vi "HFRR ADV v043.vi"() -> ()   [LabVIEW 2025] (continued)
                n2741 = Multiply(x=w3264, y=w3250) -> (x*y=w3256:dbl)
                n2742 = Subtract(x=w3257, y=w3267) -> (x-y=w3259:dbl)
                n2743 = local read "Save"() -> (w3260:bool)
                n2744 = Add(x=w3259, y=w3256) -> (x+y=w3243:dbl)
                "Elapsed time 3" <- w3243
                n2745 = And(x=w3245, y=w3260) -> (x .and. y?=w3258:bool)
                n2746 = Divide(x=w3243, y=60.0) -> (x/y=w3254:dbl)
                n2747 = local read "Test \nStatus"() -> (w3244:bool)
                n2748 = local read "clk"() -> (w3251:dbl)
                n2749 = Equal?(x=w3251, y=10.0) -> (x = y?=w3253:bool)
                n2750 = case shown="True" w3258 {
                  tunnel: w3257 -> [_ w3384]
                  tunnel: [FALSE ("Boolean 2") TRUE ("Boolean 2")] -> _
                  frame False {
                  }
                  frame True {
                    w3338 = ";" ("Substring")
                    # "Pid out/\nFreq response value"
                    n2751 = local write "act save time"(w3384) -> ()
                    n2752 = local read "FILE"() -> (w3332:string)
                    n2753 = call "file check.vi"("file name in"=w3332) -> ("error out"=w3335:errorcluster, "file name out"=w3330:string)  [unwired: 9 in]
                    n2754 = local read "LVDT STROKE"() -> (w3327:dbl)
                    n2755 = local read "Add up Stroke"() -> (w3325:dbl)
                    n2756 = call "FILE PATH CREATION.vi"("error in"=w3335, "FILE NAME :"=w3330) -> ("FILE OUT"=w3333:path)  [unwired: 8 in, 1 out]
                    n2757 = local read "STROKE Initialize"() -> (w3320:bool)
                    n2758 = Concatenate Strings(w3330, ".dgf" ("Substring")) -> (w3334:string)
                    n2759 = Subtract(x=w3327, y=w3325) -> (x-y=w3326:dbl)
                    n2760 = Absolute Value(x=w3326) -> (abs(x)=w3323:dbl)
                    n2761 = local read "FF 2"() -> (→"Frictional Force ( N )" →"Frictional Force ( N )":dbl)
                    n2762 = Build Path(base path=w3333, name or relative path=w3334) -> (appended path=w3329:path)
                    n2763 = flat-sequence {
                      tunnel: w3323 -> [w3389]
                      tunnel: [w3388] -> w3321
                      tunnel: w3320 -> [w3386]
                      tunnel: [w3391] -> w3322
                      tunnel: w3321 -> [w3391]
                      frame #0 {
                        n2764 = call <vilib>:"Mean PtByPt.vi"("x"=w3389, "sample length"="STROKE FILTER", "initialize"=w3386) -> ("mean"=w3388:dbl)  [unwired: 1 in, 1 out]
                      }
                      frame #1 {
                        "STROKE Initialize" <- FALSE ("STROKE Initialize")
                      }
                    }
                    n2765 = local read "COF 2"() -> (w3343:dbl)
                    "Coefficient of Friction" <- w3343
                    "COF 4" <- w3343
                    "Coefficient of Friction" <- w3343
                    n2766 = local read "TEMP"() -> (w3346:dbl)
                    "Temperature ( Deg C )" <- w3346
                    n2767 = local read "Humidity ( %RH )"() -> (w3345:dbl)
                    n2768 = local read "Frequency ( Hz )"() -> (w3352:dbl)
                    n2769 = local read "LVDT STROKE DISPLAY"() -> (w3324:dbl)
                    n2770 = local read "Elapsed time"() -> (w3377:dbl)
                    n2771 = local read "AIR TEMP"() -> (w3350:dbl)
                    n2772 = local read "PID-out"() -> (w3355:dbl)
                    n2773 = local write "Temperature ( Deg C )"(w3346) -> ()
                    n2774 = Number To Fractional String(number=w3324, width (-)=i16 9 ("precision (6)"), precision (6)=i16 6) -> (F-format string=w3370:string)  [unwired: 1 in]
                    n2775 = Number To Fractional String(number=w3350, width (-)=i16 9 ("precision (6)"), precision (6)=i16 3) -> (F-format string=w3369:string)  [unwired: 1 in]
                    n2776 = Number To Fractional String(number=w3346, width (-)=i16 9 ("precision (6)"), precision (6)=i16 3) -> (F-format string=w3366:string)  [unwired: 1 in]
                    n2777 = Number To Fractional String(number=w3345, width (-)=i16 9 ("precision (6)"), precision (6)=i16 3) -> (F-format string=w3363:string)  [unwired: 1 in]
                    n2778 = Number To Fractional String(number=0.0, width (-)=i16 9 ("precision (6)"), precision (6)=i16 3) -> (F-format string=w3360:string)  [unwired: 1 in]
                    n2779 = Number To Fractional String(number=w3355, width (-)=i16 9 ("precision (6)"), precision (6)=i16 3) -> (F-format string=w3356:string)  [unwired: 1 in]
                    n2780 = Number To Fractional String(number=w3352, width (-)=i16 9 ("precision (6)"), precision (6)=i16 3) -> (F-format string=w3351:string)  [unwired: 1 in]
                    n2781 = Number To Fractional String(number=w3343, width (-)=i16 9 ("precision (6)"), precision (6)=i16 6) -> (F-format string=w3378:string)  [unwired: 1 in]
                    n2782 = Number To Fractional String(number=w3377, width (-)=i16 14 ("precision (6)"), precision (6)=i16 3) -> (F-format string=w3379:string)  [unwired: 1 in]
                    n2783 = Bundle("y"=1.02, "LVDT STROKE DISPLAY"=w3324, "y"=0.98) -> (w3344:T30)  [unwired: 1 in]
                    n2784 = Number To Fractional String(number="Ambient Humidity :", width (-)=i16 9 ("precision (6)"), precision (6)=i16 6) -> (F-format string=w3336:string)  [unwired: 1 in]
                    n2785 = local read "RUN"() -> (w3342:bool)
                    n2786 = case shown="True" w3342 {
                      tunnel: w3344 -> [_ w3395]
                      tunnel: w3324 -> [_ w3394]
                      tunnel: w3324 -> [_ w3392]
                      tunnel: w3324 -> [_ w3393]
                      frame False {
                      }
                      frame True {
                        "Stroke ( mm )" <- w3395
                        "Stroke ( mm )" <- w3395
                        "Stroke 4" <- w3394
                        "Stroke 3" <- w3392
                        "Stroke 2" <- w3393
                        "measured_stroke" <- w3392
                      }
                    }
                    n2787 = Concatenate Strings(w3379, w3338, w3378, w3338, w3370, w3338, w3369, w3338, w3366, w3338, w3363, w3338, w3360, w3338, w3356, w3338, w3351, w3338, w3336, "\r") -> (w3376:string)
                    n2788 = call <vilib>:"Write Characters To File.vi"("append to file? (new file:F)"=TRUE, "character string"=w3376, "file path (dialog if empty)"=w3329) -> ()  [unwired: 2 in, 1 out]
                    "refresh flag" <- TRUE ("refresh flag")
                    "LVDT STROKE Actual" <- w3322
                  }
                }
                n2789 = case shown="True" w3244 {
                  tunnel: w3254 -> [_ w3280]
                  tunnel: w3259 -> [_ w3290]
                  tunnel: [0.0 w3286] -> _
                  tunnel: w3253 -> [_ w3285]
                  tunnel: [0.0 w3284] -> _
                  tunnel: w3243 -> [_ w3284]
                  tunnel: w3257 -> [w3273 _]
                  frame False {
                    n2790 = local write "acq timer"(w3273) -> ()
                    n2791 = local write "Test Duration Status"(0.0 ("Test Duration Status")) -> ()
                  }
                  frame True {
                    n2792 = local read "Set Hz"() -> (w3287:dbl)
                    n2793 = local write "Elapsed time"(w3280) -> ()
                    n2794 = local read "test time"() -> (w3279:dbl)
                    n2795 = Multiply(x=w3290, y=w3287) -> (x*y=w3289:dbl)
                    n2796 = case shown="False" w3285 {
                      tunnel: w3289 -> [w3291 _]
                      tunnel: [w3291 1.0] -> w3286
                      frame False {
                        n2797 = local write "Cycles elapsed"(w3291) -> ()
                      }
                      frame True {
                      }
                    }
                    n2798 = Greater?(x=w3280, y=w3279) -> (0:w3288:bool)
                    n2799 = Subtract(x=w3279, y=w3280) -> (x-y=w3278:dbl)
                    n2800 = Multiply(x=w3278, y=60.0) -> (x*y=w3277:dbl)
                    n2801 = local write "Time Remaining"(w3277) -> ()
                    n2802 = local write "Remaining Time"(w3277) -> ()
                    n2803 = case shown="True" w3288 {
                      frame False {
                      }
                      frame True {
                        n2804 = stacked-sequence {
                          frame #0 {
                            w3296 = T19."Enabled" ("Disabled")
                            w3295 = FALSE ("TEST FILE NAM,E SAVED")
                            w3297 = "" ("FILE")
                            w3298 = TRUE ("Visible")
                            n2805 = local write "Humidity"(FALSE ("Humidity")) -> ()
                            n2806 = local write "RUN"(FALSE ("OK Button 2")) -> ()
                            n2807 = local write "Heater Button"(FALSE ("Heater Button")) -> ()
                            n2808 = local write "Auto Start Test"(FALSE ("Auto Start Test")) -> ()
                            n2809 = local write "TestCompFlg"(TRUE ("StpFlg")) -> ()
                            n2810 = local read "Humidity ( %RH )"() -> (→"Rh After":dbl)
                            n2811 = property on="STOP 2" class="Bool (strict)"("Disabled"=u8 0) -> ()  [unwired: 2 in, 2 out]
                            n2812 = local read "EVENT LOG"() -> (w3303:string)
                            n2813 = call "Event Log.vi"("Content"="Test Completed", "EVENT LOG"=w3303) -> ("EVENT LOG"=w3302:string)  [unwired: 8 in, 1 out]
                            n2814 = property on="RUN" class="Bool (strict)"("Visible"=w3298) -> ()  [unwired: 2 in, 2 out]
                            n2815 = property on="Auto Start Test" class="Bool (strict)"("Visible"=w3298) -> ()  [unwired: 2 in, 2 out]
                            n2816 = local write "Batch Ref Num :"(w3297) -> ()
                            n2817 = local write "FILE"(w3297) -> ()
                            n2818 = local write "EVENT LOG"(w3302) -> ()
                            n2819 = local write "TEST FILE NAM,E SAVED"(w3295) -> ()
                            n2820 = local write "Fuel Discription :"(w3297) -> ()
                            n2821 = local write "START TEMP"(w3295) -> ()
                            n2822 = local write "Remarks :"(w3297) -> ()
                            n2823 = local write "Main Dashboard Buttons"(T1."Imaging" ("Main Dashboard Buttons")) -> ()
                            n2824 = local write "Main Tab"(T2."Adv Scar" ("Main Tab")) -> ()
                            n2825 = property on="FRICVALZ 2" class="Bool (strict)"("DisabledEnum"=w3296) -> ()  [unwired: 2 in, 2 out]
                            n2826 = property on="FRICVALZ 3" class="Bool (strict)"("DisabledEnum"=w3296) -> ()  [unwired: 2 in, 2 out]
                            n2827 = property on="FRICVALZ 4" class="Bool (strict)"("DisabledEnum"=w3296) -> ()  [unwired: 2 in, 2 out]
                          }
                          frame #1 {
                            n2828 = Wait (ms)(milliseconds to wait=u32 2000) -> ()  [unwired: 1 out]
                          }
                          frame #2 {
                            n2829 = local write "Due Write"("VC;0") -> ()
                          }
                          frame #3 {
                            n2830 = Wait (ms)(milliseconds to wait=u32 2000) -> ()  [unwired: 1 out]
                          }
                          frame #4 {
                            n2831 = local write "Due Write"("VC;0") -> ()
                          }
                          frame #5 {
                            n2832 = Wait (ms)(milliseconds to wait=u32 2000) -> ()  [unwired: 1 out]
                          }
                          frame #6 {
                            n2833 = local write "Due Write"("ST;0") -> ()
                          }
                          frame #7 {
                            n2834 = local write "measured_stroke"(0.0 ("measured_stroke")) -> ()
                            n2835 = Wait (ms)(milliseconds to wait=u32 1500) -> ()  [unwired: 1 out]
                          }
                          frame #8 {
                            n2836 = local write "Due Write"("HE;0") -> ()
                            n2837 = local write "Humidity 2"(TRUE ("Humidity")) -> ()
                          }
                        }
                      }
                    }
                    n2838 = Divide(x=w3280, y=w3279) -> (x/y=w3283:dbl)
                    n2839 = Multiply(x=w3283, y=100.0) -> (x*y=w3281:dbl)
                    n2840 = local write "Test Duration Status"(w3281) -> ()
                  }
                }
              }
              frame #2 {
                n2841 = case shown="True" "Heater Button" {
                  tunnel: [0.0 ("output") w3418] -> w3396
                  frame False {
                    w3399 = TRUE ("tmpchk")
                    n2842 = local read "TEMP"() -> (w3400:dbl)
                    n2843 = local write "Temp ini"(w3400) -> ()
                    n2844 = local write "Reset 4"(w3399) -> ()
                    n2845 = local write "tmpchk"(w3399) -> ()
                    n2846 = local write "reinit"(TRUE ("reinit")) -> ()
                    n2847 = local write "manual temp log"(TRUE ("manual temp log")) -> ()
                  }
                  frame True {
                    # "Logic to turn off\nthe heater when \ntemp is not rising.\nTime - 60 sec\nDelta t- 5°c"
                    n2848 = local read "Temp ini"() -> (w3407:dbl)
                    n2849 = local read "Auto Start Test"() -> (w3403:bool)
                    n2850 = Less?(x=w3407, y=53.0) -> (x < y?=w3405:bool)
                    n2851 = case shown="False" w3403 {
                      frame False {
                        n2852 = local read "Set Temp"() -> (w3427:dbl)
                        n2853 = local read "TEMP"() -> (w3426:dbl)
                        n2854 = Subtract(x=w3427, y=w3426) -> (x-y=w3425:dbl)
                        n2855 = Absolute Value(x=w3425) -> (abs(x)=w3424:dbl)
                        n2856 = Less?(x=w3424, y=0.5) -> (x < y?=w3422:bool)
                        n2857 = case shown="True" w3422 {
                          tunnel: "manual temp log" -> [_ w3428]
                          frame False {
                          }
                          frame True {
                            n2858 = case shown="True" w3428 {
                              selector: w3428 -> [_ w3429]
                              frame False {
                              }
                              frame True {
                                # "#Event log"
                                n2859 = Not(x=w3429) -> (.not. x?=w3430:bool)
                                n2860 = local write "manual temp log"(w3430) -> ()
                                n2861 = local read "EVENT LOG"() -> (w3433:string)
                                n2862 = call "Event Log.vi"("Content"="Target Temperature reached", "EVENT LOG"=w3433) -> ("EVENT LOG"=w3432:string)  [unwired: 8 in, 1 out]
                                n2863 = local write "EVENT LOG"(w3432) -> ()
                              }
                            }
                          }
                        }
                      }
                      frame True {
                        n2864 = local write "manual temp log"(TRUE ("manual temp log")) -> ()
                      }
                    }
                    n2865 = And(x="tmpchk", y=w3405) -> (x .and. y?=w3408:bool)
                    n2866 = case shown="True" w3408 {
                      frame False {
                      }
                      frame True {
                        n2867 = call "Elapsed Time8"("Time Target (s)"=300.0, "Reset"="Reset 4") -> ("Time has Elapsed"=w3435:bool)  [unwired: 10 in, 7 out]
                        n2868 = flat-sequence {
                          tunnel: w3435 -> [_]
                          frame #0 {
                            n2869 = local write "Reset 4"(FALSE ("Reset 4")) -> ()
                          }
                        }
                        n2870 = case shown="True" w3435 {
                          frame False {
                          }
                          frame True {
                            n2871 = local read "Temp ini"() -> (w3442:dbl)
                            n2872 = Add(x=w3442, y=5.0) -> (x+y=w3440:dbl)
                            n2873 = local read "TEMP"() -> (w3443:dbl)
                            n2874 = Greater?(x=w3443, y=w3440) -> (0:w3441:bool)
                            n2875 = case shown="False" w3441 {
                              frame False {
                                n2876 = local write "Heater Button"(FALSE ("Heater Button")) -> ()
                              }
                              frame True {
                                n2877 = local write "tmpchk"(FALSE ("tmpchk")) -> ()
                              }
                            }
                          }
                        }
                      }
                    }
                    n2878 = local read "Set Temp"() -> (w3416:dbl)
                    n2879 = local read "TEMP"() -> (w3410:dbl)
                    n2880 = call-poly <vilib>:"PID.vi"("reinitialize? (F)"="reinit", "dt (s)"=-1.0, "process variable"=w3410, "setpoint"=w3416) -> ("output"=w3413:dbl)  [unwired: 6 in, 1 out]
                    n2881 = Subtract(x=w3416, y=w3410) -> (x-y=w3417:dbl)
                    n2882 = Add(x=w3416, y=0.5) -> (x+y=w3414:dbl)
                    n2883 = Greater Or Equal?(x=w3410, y=w3414) -> ()  [unwired: 1 out]
                    n2884 = Select(t=0.0, s=FALSE, f=w3413) -> (s? t:f=w3412:dbl)
                    "PID output" <- w3412
                    n2885 = flat-sequence {
                      tunnel: w3412 -> [w3446]
                      tunnel: [w3446] -> w3418
                      frame #0 {
                        n2886 = local write "reinit"(FALSE ("reinit")) -> ()
                      }
                    }
                    n2887 = Bundle(w3417, "output"=w3412, "TEMP"=w3410) -> ()  [unwired: 1 in, 1 out]
                  }
                }
                "PID-out" <- w3396
              }
              frame #3 {
                n2888 = local read "TEMP"() -> (w3448:dbl)
                n2889 = Greater Or Equal?(x=w3448, y="Set Temp 2") -> (x >= y?=w3453:bool)
                n2890 = case shown="True" w3453 {
                  tunnel: [FALSE TRUE] -> w3451
                  frame False {
                  }
                  frame True {
                  }
                }
                "Status 13" <- w3451
                n2891 = And(x=w3451, y="trip1 8") -> (x .and. y?=w3450:bool)
                n2892 = case shown="True" w3450 {
                  frame False {
                    n2893 = local write "Heater Trip Temp"(TRUE ("Heater Trip Temp")) -> ()
                  }
                  frame True {
                    w3456 = FALSE ("OK Button 2")
                    n2894 = case shown="True" "Heater Trip Temp" {
                      selector: "Heater Trip Temp" -> [_ w3458]
                      frame False {
                      }
                      frame True {
                        n2895 = Not(x=w3458) -> (.not. x?=w3457:bool)
                        n2896 = local read "EVENT LOG"() -> (w3461:string)
                        n2897 = local write "Heater Trip Temp"(w3457) -> ()
                        n2898 = call "Event Log.vi"("Content"="Heater Trip", "EVENT LOG"=w3461) -> ("EVENT LOG"=w3460:string)  [unwired: 8 in, 1 out]
                        n2899 = local write "EVENT LOG"(w3460) -> ()
                      }
                    }
                    n2900 = local write "RUN"(w3456) -> ()
                    n2901 = property on="Auto Start Test" class="Bool (strict)"("Value"=w3456) -> ()  [unwired: 2 in, 2 out]
                    n2902 = local write "Heater Button"(w3456) -> ()
                  }
                }
              }
            }
            n2903 = case shown="False" w3167 {
              frame False {
                n2904 = disable-structure shown="Disabled" {
                  frame Disabled {
                    n2905 = stacked-sequence {
                      frame #0 {
                        n2906 = local write "RUN"(FALSE ("OK Button 2")) -> ()
                      }
                      frame #1 {
                      }
                    }
                  }
                  frame Enabled {
                  }
                }
              }
              frame True {
              }
            }
          }
        }
        n2907 = local read "Reset Graph"() -> (w3064:bool)
        n2908 = case shown="True" w3064 {
          selector: w3064 -> [_ w3081]
          frame False {
          }
          frame True {
            w3095 = 0.0 ("X Scale.Range:Maximum")
            n2909 = Not(x=w3081) -> (.not. x?=w3080:bool)
            n2910 = local write "Reset Graph"(w3080) -> ()
            n2911 = property on="Electrical Contact Resistance ( % )" class="WFChart (strict)"("XScale.Maximum"=600.0 ("X Scale.Range:Maximum"), "XScale.Minimum"=0.0 ("X Scale.Range:Minimum"), "YScale.Maximum"=100.0 ("Y Scale.Range:Maximum"), "YScale.Minimum"=0.0 ("Y Scale.Range:Minimum")) -> ()  [unwired: 2 in, 2 out]
            n2912 = property on="Frictional Force ( N )" class="WFChart (strict)"("XScale.Maximum"=600.0 ("X Scale.Range:Maximum"), "XScale.Minimum"=0.0 ("X Scale.Range:Minimum"), "YScale.Maximum"=100.0 ("Y Scale.Range:Maximum"), "YScale.Minimum"=0.0 ("Y Scale.Range:Minimum")) -> ()  [unwired: 2 in, 2 out]
            n2913 = property on="Temperature ( Deg C )" class="WFChart (strict)"("XScale.Maximum"=600.0 ("X Scale.Range:Maximum"), "XScale.Minimum"=0.0 ("X Scale.Range:Minimum"), "YScale.Maximum"=100.0 ("Y Scale.Range:Maximum"), "YScale.Minimum"=0.0 ("Y Scale.Range:Minimum")) -> ()  [unwired: 2 in, 2 out]
            n2914 = property on="Stroke ( mm )" class="WFChart (strict)"("XScale.Maximum"=600.0 ("X Scale.Range:Maximum"), "XScale.Minimum"=0.0 ("X Scale.Range:Minimum"), "YScale.Maximum"=100.0 ("Y Scale.Range:Maximum"), "YScale.Minimum"=0.0 ("Y Scale.Range:Minimum")) -> ()  [unwired: 2 in, 2 out]
            n2915 = property on="Coefficient of Friction" class="WFChart (strict)"("XScale.Maximum"=600.0 ("X Scale.Range:Maximum"), "XScale.Minimum"=0.0 ("X Scale.Range:Minimum"), "YScale.Maximum"=100.0 ("Y Scale.Range:Maximum"), "YScale.Minimum"=0.0 ("Y Scale.Range:Minimum")) -> ()  [unwired: 2 in, 2 out]
            n2916 = property on="Electrical Contact Resistance ( % )" class="WFChart (strict)"("XScale.Minimum"=0.0 ("X Scale.Range:Minimum"), "XScale.Maximum"=600.0 ("X Scale.Range:Maximum"), "YScale.Minimum"=0.0 ("Y Scale.Range:Minimum"), "YScale.Maximum"=100.0 ("Y Scale.Range:Maximum")) -> ()  [unwired: 2 in, 2 out]
            n2917 = property on="Temperature ( Deg C )" class="WFChart (strict)"("XScale.Minimum"=0.0 ("X Scale.Range:Minimum"), "XScale.Maximum"=600.0 ("X Scale.Range:Maximum"), "YScale.Minimum"=0.0 ("Y Scale.Range:Minimum"), "YScale.Maximum"=100.0 ("Y Scale.Range:Maximum")) -> ()  [unwired: 2 in, 2 out]
            n2918 = property on="Coefficient of Friction" class="WFChart (strict)"("XScale.Minimum"=0.0 ("X Scale.Range:Minimum"), "XScale.Maximum"=600.0 ("X Scale.Range:Maximum"), "YScale.Maximum"=1.0 ("X Scale.Range:Minimum"), "YScale.Minimum"=0.0 ("X Scale.Range:Minimum")) -> ()  [unwired: 2 in, 2 out]
            n2919 = property on="Frictional Force ( N )" class="WFChart (strict)"("XScale.Maximum"=600.0 ("X Scale.Range:Maximum"), "XScale.Minimum"=w3095, "YScale.Maximum"=10.0 ("Y Scale.Range:Maximum"), "YScale.Minimum"=w3095) -> ()  [unwired: 2 in, 2 out]
            n2920 = property on="Stroke ( mm )" class="WFChart (strict)"("XScale.Maximum"=600.0 ("X Scale.Range:Maximum"), "XScale.Minimum"=0.0 ("X Scale.Range:Minimum"), "YScale.Maximum"=100.0 ("Y Scale.Range:Maximum"), "YScale.Minimum"=0.0 ("Y Scale.Range:Minimum")) -> ()  [unwired: 2 in, 2 out]
          }
        }
      }
      frame "Compare Files" {
        # "Elapsed time\ncof\nstroke\nAir temp\nTemp\nHumidity"
        n2921 = case shown="True" "RSTV1 2" {
          frame False {
          }
          frame True {
            n2922 = property on="Humidity ( %RH )" class="XYGraph (strict)"("Y Scale.Display Format:Precision"=u8 0 ("Y Scale.Format & Precision:Precision")) -> ()  [unwired: 2 in, 2 out]
            n2923 = property on="Humidity ( %RH )" class="XYGraph (strict)"("X Scale.Range:Minimum"=0.0, "X Scale.Range:Maximum"=75.0, "Y Scale.Range:Minimum"=48.0, "Y Scale.Range:Maximum"=58.0) -> ()  [unwired: 2 in, 2 out]
          }
        }
        n2924 = case shown="True" "RST CP 2" {
          frame False {
          }
          frame True {
            n2925 = property on="XY Graph 13" class="XYGraph (strict)"("Y Scale.Display Format:Precision"=u8 0 ("Y Scale.Format & Precision:Precision")) -> ()  [unwired: 2 in, 2 out]
            n2926 = property on="XY Graph 13" class="XYGraph (strict)"("X Scale.Range:Minimum"=0.0, "X Scale.Range:Maximum"=75.0, "Y Scale.Range:Minimum"=0.0, "Y Scale.Range:Maximum"=100.0) -> ()  [unwired: 2 in, 2 out]
          }
        }
        n2927 = case shown="True" "RST CP" {
          frame False {
          }
          frame True {
            n2928 = property on="Sample Temperature ( °C )" class="XYGraph (strict)"("Y Scale.Display Format:Precision"=u8 2 ("Y Scale.Format & Precision:Precision")) -> ()  [unwired: 2 in, 2 out]
            n2929 = property on="Sample Temperature ( °C )" class="XYGraph (strict)"("X Scale.Range:Minimum"=0.0, "X Scale.Range:Maximum"=75.0, "Y Scale.Range:Minimum"=58.0, "Y Scale.Range:Maximum"=62.0) -> ()  [unwired: 2 in, 2 out]
          }
        }
        n2930 = case shown="True" "RSTV1 3" {
          frame False {
          }
          frame True {
            n2931 = property on="Air Temperature  ( °C )" class="XYGraph (strict)"("Y Scale.Display Format:Precision"=u8 2 ("Y Scale.Format & Precision:Precision")) -> ()  [unwired: 2 in, 2 out]
            n2932 = property on="Air Temperature  ( °C )" class="XYGraph (strict)"("X Scale.Range:Minimum"=0.0 ("Y Scale.Range:Minimum"), "X Scale.Range:Maximum"=75.0 ("Y Scale.Range:Maximum"), "Y Scale.Range:Minimum"=20.0 ("X Scale.Range:Minimum"), "Y Scale.Range:Maximum"=26.0 ("X Scale.Range:Maximum")) -> ()  [unwired: 2 in, 2 out]
          }
        }
        n2933 = case shown="True" "RSTV1 4" {
          frame False {
          }
          frame True {
            n2934 = property on="Stroke ( mm )" class="XYGraph (strict)"("Y Scale.Display Format:Precision"=u8 2 ("Y Scale.Format & Precision:Precision")) -> ()  [unwired: 2 in, 2 out]
            n2935 = property on="Stroke ( mm )" class="XYGraph (strict)"("X Scale.Range:Minimum"=0.0 ("Y Scale.Range:Maximum"), "X Scale.Range:Maximum"=75.0 ("X Scale.Range:Minimum"), "Y Scale.Range:Minimum"=0.98, "Y Scale.Range:Maximum"=1.02) -> ()  [unwired: 2 in, 2 out]
          }
        }
        n2936 = case shown="True" "rstv2" {
          frame False {
          }
          frame True {
            n2937 = property on="Coefficient Of Friction" class="XYGraph (strict)"("Y Scale.Display Format:Precision"=u8 3 ("Y Scale.Format & Precision:Precision")) -> ()  [unwired: 2 in, 2 out]
            n2938 = property on="Coefficient Of Friction" class="XYGraph (strict)"("X Scale.Range:Minimum"=0.0 ("Y Scale.Range:Maximum"), "X Scale.Range:Maximum"=75.0, "Y Scale.Range:Minimum"=0.0, "Y Scale.Range:Maximum"=1.0 ("X Scale.Range:Minimum")) -> ()  [unwired: 2 in, 2 out]
          }
        }
        n2939 = case shown="True" "RST CP 3" {
          frame False {
          }
          frame True {
            n2940 = property on="Air Temp ( °C ) vs Humidity ( % RH )" class="XYGraph (strict)"("X Scale.Range:Minimum"=18.0, "X Scale.Range:Maximum"=28.0 ("X Scale.Range:Minimum"), "Y Scale.Range:Minimum"=30.0 ("X Scale.Range:Minimum"), "Y Scale.Range:Maximum"=70.0 ("X Scale.Range:Minimum")) -> ()  [unwired: 2 in, 2 out]
          }
        }
        n2941 = case shown="True" "OPEN 1" {
          frame False {
          }
          frame True {
            (unwired) 0  # existing file
            w3737 = "Choose a datalog file to open"  # prompt
            n2942 = local write "OPEN 1"(FALSE ("OPEN 1")) -> ()
            n2943 = String To Path(string="C:\\LAB-IQ\\Data\\") -> (path=w3722:path)
            n2944 = File Dialog(6:"*.dgf" ("pattern"), 7:w3737, 11:w3722) -> (0:w3720:errorcluster, 3:w3728:path)  [unwired: 4 in, 2 out]
            n2945 = Unbundle(w3720) -> ()  [unwired: 3 out]
            n2946 = Strip Path(path=w3728) -> (name=w3727:string)  [unwired: 1 out]
            n2947 = Path To String(path=w3728) -> (string=w3723:string)
            "string1" <- w3723
            n2948 = Match Pattern(string=w3727, regular expression=".dgf") -> (before substring=→"String Control":string)  [unwired: 1 in, 3 out]
            n2949 = Match Pattern(string=w3723, regular expression=".dgf" ("substring (\"\")")) -> (before substring=w3733:string)  [unwired: 1 in, 3 out]
            n2950 = Concatenate Strings(w3733, ".duf" ("Substring")) -> (w3729:string)
            n2951 = String To Path(string=w3729) -> (path=w3734:path)
            n2952 = call <vilib>:"Read Characters From File.vi"("file path (dialog if empty)"=w3734, "start of read offset (chars.:0)"=60 ("start of read offset (chars.: 0)")) -> ("character string"=→"String Control 2":string)  [unwired: 4 in, 3 out]
          }
        }
        n2953 = case shown="True" "OPEN 2" {
          frame False {
          }
          frame True {
            (unwired) 0  # existing file
            w3755 = "Choose a datalog file to open"  # prompt
            n2954 = local write "OPEN 2"(FALSE ("OPEN 1")) -> ()
            n2955 = String To Path(string="C:\\LAB-IQ\\Data\\") -> (path=w3740:path)
            n2956 = File Dialog(6:"*.dgf" ("pattern"), 7:w3755, 11:w3740) -> (0:w3738:errorcluster, 3:w3746:path)  [unwired: 4 in, 2 out]
            n2957 = Unbundle(w3738) -> ()  [unwired: 3 out]
            n2958 = Strip Path(path=w3746) -> (name=w3744:string)  [unwired: 1 out]
            n2959 = Path To String(path=w3746) -> (string=w3741:string)
            "string1 2" <- w3741
            n2960 = Match Pattern(string=w3744, regular expression=".dgf") -> (before substring=→"String Control 3":string)  [unwired: 1 in, 3 out]
            n2961 = Match Pattern(string=w3741, regular expression=".dgf" ("substring (\"\")")) -> (before substring=w3752:string)  [unwired: 1 in, 3 out]
            n2962 = Concatenate Strings(w3752, ".duf" ("Substring")) -> (w3749:string)
            n2963 = String To Path(string=w3749) -> (path=w3747:path)
            n2964 = call <vilib>:"Read Characters From File.vi"("file path (dialog if empty)"=w3747, "start of read offset (chars.:0)"=60 ("start of read offset (chars.: 0)")) -> ("character string"=→"String Control 4":string)  [unwired: 4 in, 3 out]
          }
        }
        n2965 = case shown="True" "OPEN 3" {
          frame False {
          }
          frame True {
            (unwired) 0  # existing file
            w3773 = "Choose a datalog file to open"  # prompt
            n2966 = local write "OPEN 3"(FALSE ("OPEN 1")) -> ()
            n2967 = String To Path(string="C:\\LAB-IQ\\Data\\") -> (path=w3758:path)
            n2968 = File Dialog(6:"*.dgf" ("pattern"), 7:w3773, 11:w3758) -> (0:w3756:errorcluster, 3:w3764:path)  [unwired: 4 in, 2 out]
            n2969 = Unbundle(w3756) -> ()  [unwired: 3 out]
            n2970 = Strip Path(path=w3764) -> (name=w3762:string)  [unwired: 1 out]
            n2971 = Path To String(path=w3764) -> (string=w3759:string)
            "string1 3" <- w3759
            n2972 = Match Pattern(string=w3762, regular expression=".dgf") -> (before substring=→"String Control 5":string)  [unwired: 1 in, 3 out]
            n2973 = Match Pattern(string=w3759, regular expression=".dgf" ("substring (\"\")")) -> (before substring=w3769:string)  [unwired: 1 in, 3 out]
            n2974 = Concatenate Strings(w3769, ".duf" ("Substring")) -> (w3766:string)
            n2975 = String To Path(string=w3766) -> (path=w3770:path)
            n2976 = call <vilib>:"Read Characters From File.vi"("file path (dialog if empty)"=w3770, "start of read offset (chars.:0)"=60 ("start of read offset (chars.: 0)")) -> ("character string"=→"String Control 6":string)  [unwired: 4 in, 3 out]
          }
        }
        n2977 = case shown="True" "OPEN 4" {
          frame False {
          }
          frame True {
            (unwired) 0  # existing file
            w3791 = "Choose a datalog file to open"  # prompt
            n2978 = local write "OPEN 4"(FALSE ("OPEN 1")) -> ()
            n2979 = String To Path(string="C:\\LAB-IQ\\Data\\") -> (path=w3776:path)
            n2980 = File Dialog(6:"*.dgf" ("pattern"), 7:w3791, 11:w3776) -> (0:w3774:errorcluster, 3:w3782:path)  [unwired: 4 in, 2 out]
            n2981 = Unbundle(w3774) -> ()  [unwired: 3 out]
            n2982 = Strip Path(path=w3782) -> (name=w3780:string)  [unwired: 1 out]
            n2983 = Path To String(path=w3782) -> (string=w3777:string)
            "string1 4" <- w3777
            n2984 = Match Pattern(string=w3780, regular expression=".dgf") -> (before substring=→"String Control 7":string)  [unwired: 1 in, 3 out]
            n2985 = Match Pattern(string=w3777, regular expression=".dgf" ("substring (\"\")")) -> (before substring=w3787:string)  [unwired: 1 in, 3 out]
            n2986 = Concatenate Strings(w3787, ".duf" ("Substring")) -> (w3784:string)
            n2987 = String To Path(string=w3784) -> (path=w3788:path)
            n2988 = call <vilib>:"Read Characters From File.vi"("file path (dialog if empty)"=w3788, "start of read offset (chars.:0)"=60 ("start of read offset (chars.: 0)")) -> ("character string"=→"String Control 8":string)  [unwired: 4 in, 3 out]
          }
        }
      }
      frame "About" {
        # "Elapsed time\ncof\nstroke\nmean pos\nTemp\nHumidity"
        n2989 = disable-structure shown="Disabled" {
          frame Disabled {
            n2990 = case shown="True" "Export" {
              frame False {
              }
              frame True {
                w3813 = "                                      " ("string")
                w3815 = "\r"
                (unwired) i16 6 ("width (-)")
                w3892 = "\r"
                w3824 = "\r"
                n2991 = local write "Export"(FALSE ("Export")) -> ()
                n2992 = local read "String 29"() -> (w3861:string)
                n2993 = local read "String 34"() -> (w3849:string)
                n2994 = local read "String 35"() -> (w3844:string)
                n2995 = local read "String 37"() -> (w3840:string)
                n2996 = local read "String 36"() -> (w3837:string)
                n2997 = local read "String 38"() -> (w3834:string)
                n2998 = local read "String 39"() -> (w3831:string)
                n2999 = Match Pattern(string=w3861, regular expression=".dwm") -> (before substring=w3857:string)  [unwired: 1 in, 3 out]
                "before substring" <- w3857
                n3000 = local read "S 38"() -> (w3852:string)
                n3001 = local read "S 39"() -> (w3845:string)
                n3002 = local read "Temperature before test 2"() -> (w3881:dbl)
                n3003 = local read "Temperature after test 2"() -> (w3886:dbl)
                n3004 = local read "Humidity before test 2"() -> (w3867:dbl)
                n3005 = local read "Humidity after test 2"() -> (w3882:dbl)
                n3006 = local read "MWSD 2"() -> (w3878:dbl)
                n3007 = local read "WS1.4 2"() -> (w3894:dbl)
                n3008 = local read "HCF 2"() -> (w3890:dbl)
                n3009 = local read "AVP 2"() -> (w3879:dbl)
                n3010 = Concatenate Strings("1," ("string"), w3852) -> (w3851:string)
                n3011 = Concatenate Strings("2," ("string"), w3849) -> (w3848:string)
                n3012 = Concatenate Strings("3," ("string"), w3845) -> (w3847:string)
                n3013 = Concatenate Strings("4," ("string"), w3844) -> (w3843:string)
                n3014 = Concatenate Strings("5," ("string"), w3840) -> (w3841:string)
                n3015 = Concatenate Strings("6," ("string"), w3837) -> (w3838:string)
                n3016 = Concatenate Strings("7," ("string"), w3834) -> (w3835:string)
                n3017 = Concatenate Strings("8," ("string"), w3831) -> (w3832:string)
                n3018 = local read "Sample ID"() -> (w3899:string)
                n3019 = case shown="\"xlx\"" "Select File Type" {
                  tunnel: w3857 -> [w3902 w3904 w3906]
                  tunnel: [w3900 w3905 w3907] -> w3856
                  frame "xlx" {
                    n3020 = Concatenate Strings(w3902, ".xls" ("string")) -> (w3900:string)
                  }
                  frame "csv" {
                    n3021 = Concatenate Strings(w3904, ".csv" ("string")) -> (w3905:string)
                  }
                  frame "txt" {
                    n3022 = Concatenate Strings(w3906, ".txt" ("string")) -> (w3907:string)
                  }
                }
                n3023 = local read "Test Date"() -> (w3898:string)
                n3024 = local read "String 45"() -> (w3812:string)
                n3025 = local read "String 31"() -> (w3897:string)
                n3026 = local read "String 32"() -> (w3896:string)
                n3027 = local read "TITTLE"() -> (w3820:string)
                n3028 = Number To Fractional String(number=w3867, width (-)=i16 6, precision (6)=i16 2) -> (F-format string=w3866:string)  [unwired: 1 in]
                n3029 = Number To Fractional String(number=w3881, width (-)=i16 6, precision (6)=i16 2) -> (F-format string=w3887:string)  [unwired: 1 in]
                n3030 = Number To Fractional String(number=w3882, width (-)=i16 6, precision (6)=i16 2) -> (F-format string=w3880:string)  [unwired: 1 in]
                n3031 = Number To Fractional String(number=w3886, width (-)=i16 6, precision (6)=i16 2) -> (F-format string=w3885:string)  [unwired: 1 in]
                n3032 = Number To Fractional String(number=w3878, width (-)=i16 6, precision (6)=i16 2) -> (F-format string=w3876:string)  [unwired: 1 in]
                n3033 = Number To Fractional String(number=w3879, width (-)=i16 6, precision (6)=i16 2) -> (F-format string=w3877:string)  [unwired: 1 in]
                n3034 = Number To Fractional String(number=w3890, width (-)=i16 6, precision (6)=i16 2) -> (F-format string=w3891:string)  [unwired: 1 in]
                n3035 = Number To Fractional String(number=w3894, precision (6)=i16 2) -> (F-format string=w3895:string)  [unwired: 2 in]
                n3036 = local read "s.NO"() -> (w3814:string)
                n3037 = Concatenate Strings("=" ("string"), w3820) -> (w3819:string)
                n3038 = Concatenate Strings("S.No," ("string"), "                                       Parameters" ("string")) -> (w3825:string)
                n3039 = Concatenate Strings(w3892, w3851, w3866, w3892, w3848, w3887, w3892, w3847, w3880, w3892, w3843, w3885, w3892, w3841, w3876, w3892, w3838, w3877, w3892, w3835, w3891, w3892, w3832, w3895) -> (w3854:string)
                n3040 = Concatenate Strings(w3824, "," ("string"), w3812, w3814, w3813, w3896, w3899, w3813, w3897, w3898, w3824) -> (w3822:string)
                n3041 = local read "Tested by"() -> (w3828:string)
                n3042 = local read "String 33"() -> (w3829:string)
                n3043 = Concatenate Strings("," ("string"), "                                                                             " ("string")) -> (w3817:string)
                n3044 = Concatenate Strings(w3819, w3815, w3822, w3815, w3825, w3854, w3815, w3817, w3829, w3828) -> (→"export":string)
                n3045 = String To Path(string=w3856) -> (path=w3863:path)
                n3046 = local read "export"() -> (w3858:string)
                n3047 = call <vilib>:"Write Characters To File.vi"("append to file? (new file:F)"=FALSE, "character string"=w3858, "file path (dialog if empty)"=w3863) -> ()  [unwired: 2 in, 1 out]
              }
            }
          }
          frame Enabled {
          }
        }
        n3048 = case shown="True" "OK Button 17" {
          frame False {
          }
          frame True {
            (unwired) 0  # existing file
            w4116 = "Choose a datalog file to open"  # prompt
            n3049 = local write "OK Button 17"(FALSE ("OK Button 17")) -> ()
            n3050 = local read "String"() -> (w4111:string)
            n3051 = String To Path(string=w4111) -> (path=w4112:path)
            n3052 = File Dialog(6:"*.duf" ("pattern"), 7:w4116, 11:w4112) -> (0:w4103:errorcluster, 3:w4122:path)  [unwired: 4 in, 2 out]
            n3053 = Unbundle(w4103) -> ()  [unwired: 3 out]
            n3054 = Open/Create/Replace File "Open File"(file path (use dialog)=w4122) -> (refnum out=w4114:refnum<file>)  [unwired: 5 in, 2 out]
            n3055 = Strip Path(path=w4122) -> (name=w4120:string)  [unwired: 1 out]
            n3056 = Path To String(path=w4122) -> (string=w4105:string)
            n3057 = while {
              tunnel: w4114 -> [w4126]
              i -> [w4123]
              stop <- w4124 continue-if-true
              (unwired) TRUE ("line mode (F)")
              n3058 = Read from Text File "Read File"(file (use dialog)=w4126) -> (text=w4125:string)  [unwired: 3 in, 3 out]
              n3059 = local write "Numeric 16"(w4123) -> ()
              n3060 = String Length(string=w4125) -> (length=w4128:i32)
              n3061 = Greater?(x=w4128, y=1) -> (0:w4124:bool)
            }
            n3062 = local write "String 29"(w4105) -> ()
            n3063 = Search and Replace String(input string=w4105, search string=".duf", replace string=".dgf" ("replace string (\"\")")) -> (result string=→"String Indicator 4":string)  [unwired: 5 in, 3 out]
            n3064 = Match Pattern(string=w4120, regular expression=".dwm") -> (before substring=w4104:string)  [unwired: 1 in, 3 out]
            "String Indicator" <- w4104
            n3065 = Match Pattern(string=w4105, regular expression=".dwm" ("substring (\"\")")) -> (before substring=w4106:string)  [unwired: 1 in, 3 out]
            "String Indicator 3" <- w4106
            n3066 = local write "TITTLE 2"(w4104) -> ()
            n3067 = String To Path(string=w4106) -> (path=w4113:path)
            "path" <- w4113
            n3068 = call <vilib>:"Read Characters From File.vi"("file path (dialog if empty)"=w4113, "start of read offset (chars.:0)"=60 ("start of read offset (chars.: 0)")) -> ("character string"=→"String Indicator 2":string)  [unwired: 4 in, 3 out]
          }
        }
        n3069 = call <vilib>:"Query Available Printers.vi"() -> ("system configured printers"=w3805:string[])  [unwired: 9 in, 2 out]
        "System Configured Printers 2" <- w3805
        n3070 = local read "OK Button 16"() -> (w3802:bool)
        n3071 = case shown="True" "OK Button 16" {
          frame False {
          }
          frame True {
            n3072 = stacked-sequence {
              frame #0 {
                n3073 = local read "Numeric 16"() -> (w4130:i32)
                n3074 = local write "Numeric 10"(w4130) -> ()
              }
              frame #1 {
                n3075 = local read "String 29"() -> (w4133:string)
                n3076 = String To Path(string=w4133) -> (path=w4132:path)
                n3077 = Open/Create/Replace File "Open File"(file path (use dialog)=w4132) -> (refnum out=w4134:refnum<file>)  [unwired: 5 in, 2 out]
                n3078 = for {
                  N: 16 -> [_]
                  tunnel: w4134 -> [w4141]
                  i -> [w4137]
                  (unwired) TRUE ("line mode (F)")
                  n3079 = Read from Text File "Read File"(file (use dialog)=w4141) -> (text=w4135:string)  [unwired: 3 in, 3 out]
                  n3080 = Match Pattern(string=w4135, regular expression="(") -> (after substring=w4140:string)  [unwired: 1 in, 3 out]
                  n3081 = Match Pattern(string=w4140, regular expression=")") -> (before substring=w4136:string)  [unwired: 1 in, 3 out]
                  n3082 = case shown="1" w4137 {
                    tunnel: w4136 -> [w4142 w4143 _ _ w4144 w4145 w4146 w4148 w4150 w4152 w4154 w4156 w4158 w4160 _]
                    tunnel: w4135 -> [_ _ _ _ _ _ _ _ _ _ _ _ _ _ _]
                    frame 0 {
                      "TITTLE" <- w4142
                    }
                    frame 1 {
                      "Sample ID" <- w4143
                    }
                    frame 2 {
                    }
                    frame 3 {
                    }
                    frame 4 {
                      "Test Date" <- w4144
                    }
                    frame 5 {
                      "Tested by" <- w4145
                    }
                    frame 6 {
                      n3083 = Fract/Exp String To Number(string=w4146) -> (number=→"Humidity before test 2":dbl)  [unwired: 3 in, 1 out]
                    }
                    frame 7 {
                      n3084 = Fract/Exp String To Number(string=w4148) -> (number=→"Temperature before test 2":dbl)  [unwired: 3 in, 1 out]
                    }
                    frame 8 {
                      n3085 = Fract/Exp String To Number(string=w4150) -> (number=→"Humidity after test 2":dbl)  [unwired: 3 in, 1 out]
                    }
                    frame 9 {
                      n3086 = Fract/Exp String To Number(string=w4152) -> (number=→"Temperature after test 2":dbl)  [unwired: 3 in, 1 out]
                    }
                    frame 10 {
                      n3087 = Fract/Exp String To Number(string=w4154) -> (number=→"MWSD 2":dbl)  [unwired: 3 in, 1 out]
                    }
                    frame 11 {
                      n3088 = Fract/Exp String To Number(string=w4156) -> (number=→"AVP 2":dbl)  [unwired: 3 in, 1 out]
                    }
                    frame 12 {
                      n3089 = Fract/Exp String To Number(string=w4158) -> (number=→"HCF 2":dbl)  [unwired: 3 in, 1 out]
                    }
                    frame 13 {
                      n3090 = Fract/Exp String To Number(string=w4160) -> (number=→"WS1.4 2":dbl)  [unwired: 3 in, 1 out]
                    }
                    frame 14, Default {
                    }
                  }
                }
              }
              frame #2 {
              }
            }
            n3091 = local write "OK Button 16"(FALSE ("OK Button 13")) -> ()
          }
        }
        n3092 = Index Array(array=w3805, index="Select Printer 3") -> (element=w3807:string)
        "Selected Printer" <- w3807
        n3093 = case shown="True" w3802 {
          frame False {
          }
          frame True {
            n3094 = flat-sequence {
              frame #0 {
              }
              frame #1 {
                n3095 = Wait (ms)(milliseconds to wait=u32 100) -> ()  [unwired: 1 out]
              }
              frame #2 {
                n3096 = local write "OK Button 16"(FALSE ("Print 3")) -> ()
              }
            }
          }
        }
        n3097 = case shown="True" "Print" {
          tunnel: w3807 -> [_ w4099]
          frame False {
          }
          frame True {
            (unwired) i16 6 ("width (-)")
            (unwired) "TESTED BY : "
            (unwired) "TESTED DATE :"
            (unwired) "SAMPLE ID : "
            (unwired) "SAMPLE DESIGN : "
            w4057 = "\r"
            w4074 = "\r"
            # "add image"
            n3098 = local read "Sample ID"() -> (w4047:string)
            n3099 = local read "Tested by"() -> (w4050:string)
            n3100 = local read "String 34"() -> (w4037:string)
            n3101 = local read "String 45"() -> (w4017:string)
            n3102 = local read "String 35"() -> (w4032:string)
            n3103 = local read "String 37"() -> (w4030:string)
            n3104 = local read "String 32"() -> (w4052:string)
            n3105 = local read "String 36"() -> (w4027:string)
            n3106 = local read "String 31"() -> (w4051:string)
            n3107 = local read "Test Date"() -> (w4048:string)
            n3108 = local read "String 33"() -> (w4053:string)
            n3109 = local read "String 38"() -> (w4023:string)
            n3110 = local read "String 39"() -> (w4020:string)
            n3111 = local write "Print"(FALSE ("Print FF")) -> ()
            n3112 = local read "S 39"() -> (w4035:string)
            n3113 = local read "S 38"() -> (w4042:string)
            n3114 = local read "Temperature before test 2"() -> (w4073:dbl)
            n3115 = local read "Temperature after test 2"() -> (w4063:dbl)
            n3116 = local read "Humidity before test 2"() -> (w4088:dbl)
            n3117 = local read "Humidity after test 2"() -> (w4072:dbl)
            n3118 = local read "MWSD 2"() -> (w4077:dbl)
            n3119 = local read "WS1.4 2"() -> (w4055:dbl)
            n3120 = Concatenate Strings("2)" ("string"), w4037) -> (w4038:string)
            n3121 = Concatenate Strings("3)" ("string"), w4035) -> (w4036:string)
            n3122 = Concatenate Strings("1)" ("string"), w4042) -> (w4041:string)
            n3123 = Concatenate Strings("4)" ("string"), w4032) -> (w4033:string)
            n3124 = Concatenate Strings("5)" ("string"), w4030) -> (w4029:string)
            n3125 = Concatenate Strings("6)" ("string"), w4027) -> (w4026:string)
            n3126 = Concatenate Strings("7)" ("string"), w4023) -> (w4024:string)
            n3127 = Concatenate Strings("8)" ("string"), w4020) -> (w4021:string)
            n3128 = local read "HCF 2"() -> (w4059:dbl)
            n3129 = local read "AVP 2"() -> (w4076:dbl)
            n3130 = local read "s.NO"() -> (w4018:string)
            n3131 = call <vilib>:"New Report.vi"("report type"=enum16{"Standard Report", "HTML"}."Standard Report") -> ("report out"=w4097:refnum<class "NI_report.lvclass">, "error out"=w4096:errorcluster)  [unwired: 13 in]
            n3132 = local read "TITTLE"() -> (w4049:string)
            n3133 = Concatenate Strings(w4074, w4017, w4018, w4074, w4052, w4047, w4074, w4051, w4048, w4074, w4053, w4050, w4074) -> (w4067:string)
            "test by" <- w4067
            n3134 = Number To Fractional String(number=w4073, width (-)=i16 6, precision (6)=i16 2) -> (F-format string=w4062:string)  [unwired: 1 in]
            n3135 = Number To Fractional String(number=w4072, width (-)=i16 6, precision (6)=i16 2) -> (F-format string=w4075:string)  [unwired: 1 in]
            n3136 = Number To Fractional String(number=w4088, width (-)=i16 6, precision (6)=i16 2) -> (F-format string=w4093:string)  [unwired: 1 in]
            n3137 = Number To Fractional String(number=w4077, width (-)=i16 6, precision (6)=i16 2) -> (F-format string=w4079:string)  [unwired: 1 in]
            n3138 = Number To Fractional String(number=w4063, width (-)=i16 6, precision (6)=i16 2) -> (F-format string=w4064:string)  [unwired: 1 in]
            n3139 = Number To Fractional String(number=w4076, width (-)=i16 6, precision (6)=i16 2) -> (F-format string=w4078:string)  [unwired: 1 in]
            n3140 = Number To Fractional String(number=w4059, width (-)=i16 6, precision (6)=i16 2) -> (F-format string=w4058:string)  [unwired: 1 in]
            n3141 = Number To Fractional String(number=w4055, precision (6)=i16 2) -> (F-format string=w4054:string)  [unwired: 2 in]
            n3142 = call-dynamic "Set Report Header Text.vi"("report in"=w4097, "center header text"=w4049, "error in (no error)"=w4096) -> ("report out"=w4068:refnum<class "NI_report.lvclass">, "error out"=w4069:errorcluster)  [unwired: 11 in]
            n3143 = Concatenate Strings(w4057, w4041, w4093, w4057, w4038, w4062, w4057, w4036, w4075, w4057, w4033, w4064, w4057, w4029, w4079, w4057, w4026, w4078, w4057, w4024, w4058, w4057, w4021, w4054) -> (w4045:string)
            "export 2" <- w4045
            n3144 = call-poly <vilib>:"Append Report Text.vi"("report in"=w4068, "text"=w4067, "error in (no error)"=w4069) -> ("report out"=w4071:refnum<class "NI_report.lvclass">, "error out"=w4070:errorcluster)  [unwired: 9 in, 2 out]
            n3145 = local read "test by"() -> (w4044:string)
            n3146 = local read "TITTLE"() -> (w4046:string)
            n3147 = call-poly <vilib>:"Append Report Text.vi"("report in"=w4071, "error in (no error)"=w4070) -> ("report out"=w4092:refnum<class "NI_report.lvclass">, "error out"=w4090:errorcluster)  [unwired: 10 in, 2 out]
            n3148 = Concatenate Strings(w4046, w4045, w4044) -> (→"output":string)
            n3149 = call-poly <vilib>:"Append Report Text.vi"("report in"=w4092, "text"=w4045, "error in (no error)"=w4090) -> ("report out"=w4091:refnum<class "NI_report.lvclass">, "error out"=w4089:errorcluster)  [unwired: 9 in, 2 out]
            n3150 = call-dynamic "Print Report.vi"("report in"=w4091, "printer name (default)"=w4099, "error in (no error)"=w4089) -> ("report out"=w4101:refnum<class "NI_report.lvclass">, "error out"=w4102:errorcluster)  [unwired: 11 in]
            n3151 = call-dynamic "Dispose Report.vi"("report in"=w4101, "error in (no error)"=w4102) -> ()  [unwired: 13 in, 1 out]
          }
        }
        n3152 = case shown="True" "Print 2" {
          frame False {
          }
          frame True {
            n3153 = flat-sequence {
              frame #0 {
                n3154 = local read "s.NO"() -> (→"s.NO 2":string)
                n3155 = Wait (ms)(milliseconds to wait=u32 20) -> ()  [unwired: 1 out]
                n3156 = local read "Sample ID  3"() -> (→"Sample ID  6":string)
                n3157 = local read "Sample ID  4"() -> (→"Sample ID  7":string)
                n3158 = local read "Sample ID"() -> (→"Sample ID  2":string)
                n3159 = local read "Tested by"() -> (→"Tested by 2":string)
                n3160 = local read "Test Date"() -> (→"Test Date 2":string)
                n3161 = local read "Humidity after test 3"() -> (→"Humidity after test 4":dbl)
                n3162 = local read "Ref A Test Date :"() -> (→"TITTLE 4":string)
                n3163 = local read "Temperature before test 3"() -> (w3924:dbl)
                n3164 = local read "Temperature before test 3"() -> (→"Temperature after test 5":dbl)
                n3165 = local read "Temperature after test 3"() -> (→"Temperature after test 4":dbl)
                n3166 = local read "Humidity before test 3"() -> (→"Humidity before test 4":dbl)
                n3167 = local write "Temperature before test 3"(w3924) -> ()
                n3168 = local read "image data"() -> (w3915:T16)
                n3169 = String To Path(string="C:\\LAB-IQ\\im\\Temp_resized.jpg") -> (path=w3916:path)
                "path 2" <- w3916
                n3170 = call <vilib>:"Write JPEG File.vi"("image data"=w3915, "path to JPEG file"=w3916) -> ()  [unwired: 8 in, 2 out]
                "Ref A Test Date :" <- "Ref A Test Date :"
                "Ref B Test Date :" <- "Ref B Test Date :"
                "Ref B Scar Value :" <- "Ref B Scar Value :"
                "Ref A Scar Value :" <- "Ref A Scar Value :"
              }
              frame #1 {
                (unwired) HTML_Report_Image_Alignment."MIDDLE" ("alignment (default)")
                w3952 = u16 0 items=["portrait", "landscape"] ("orientation (portrait)")
                (unwired) HTML_Report_Image_Alignment."ABSMIDDLE" ("alignment (default)")
                (unwired) "TESTED BY : "
                (unwired) "TESTED DATE :"
                (unwired) "SAMPLE ID : "
                (unwired) "SAMPLE DESIGN : "
                w3985 = "\r"
                # "add image"
                n3171 = Wait (ms)(milliseconds to wait=u32 20) -> ()  [unwired: 1 out]
                n3172 = local read "Sample ID  2"() -> (w3978:string)
                n3173 = local read "Wear Scar X"() -> (w3950:dbl)
                "Length ( microns ) 2" <- w3950
                n3174 = local read "Wear Scar Y"() -> (w3949:dbl)
                "Wear Scar Y ( microns ) :" <- w3949
                n3175 = local read "Test Date 2"() -> (w3979:string)
                n3176 = local read "Tested by 2"() -> (w3980:string)
                n3177 = local read "String 46"() -> (w3976:string)
                n3178 = local read "String 48"() -> (w3982:string)
                n3179 = local read "String 47"() -> (w3981:string)
                n3180 = local read "String 49"() -> (w3983:string)
                n3181 = local read "String 10"() -> (w3936:string)
                n3182 = local read "s.NO 2"() -> (w3977:string)
                n3183 = Add(x=w3950, y=w3949) -> (x+y=w3948:dbl)
                n3184 = call <vilib>:"New Report.vi"("report type"=enum16{"Standard Report", "HTML"}."HTML") -> ("report out"=w3956:refnum<class "NI_report.lvclass">, "error out"=w3954:errorcluster)  [unwired: 13 in]
                n3185 = Concatenate Strings(w3985, w3976, w3977, w3985, w3982, w3978, w3985, w3981, w3979, w3985, w3983, w3980, w3985) -> (→"test by 2":string)
                n3186 = Concatenate Strings("C:\\LAB-IQ\\Data\\" ("string"), w3936, ".jpg" ("string")) -> ()  [unwired: 1 out]
                n3187 = Divide(x=w3948, y=2.0) -> (x/y=→"Mean Wear ( microns) :":dbl)
                n3188 = call-dynamic "Set Report Orientation.vi"("report in"=w3956, "orientation (portrait)"=w3952, "error in (no error)"=w3954) -> ("report out"=w3955:refnum<class "NI_report.lvclass">, "error out"=w3953:errorcluster)  [unwired: 11 in]
                n3189 = for {
                  N: 5 -> [_]
                  tunnel: w3955 -> [w4006]
                  tunnel: [w4005] -> w3934
                  tunnel: w3953 -> [w4004]
                  tunnel: [w4003] -> w3933